vi "Splash screen.vi"(8 "error in (no error)":errorcluster) -> (0 "error out":errorcluster)   [LabVIEW 2016]
panel:
  out "String":string
  in  "Blank Button":bool
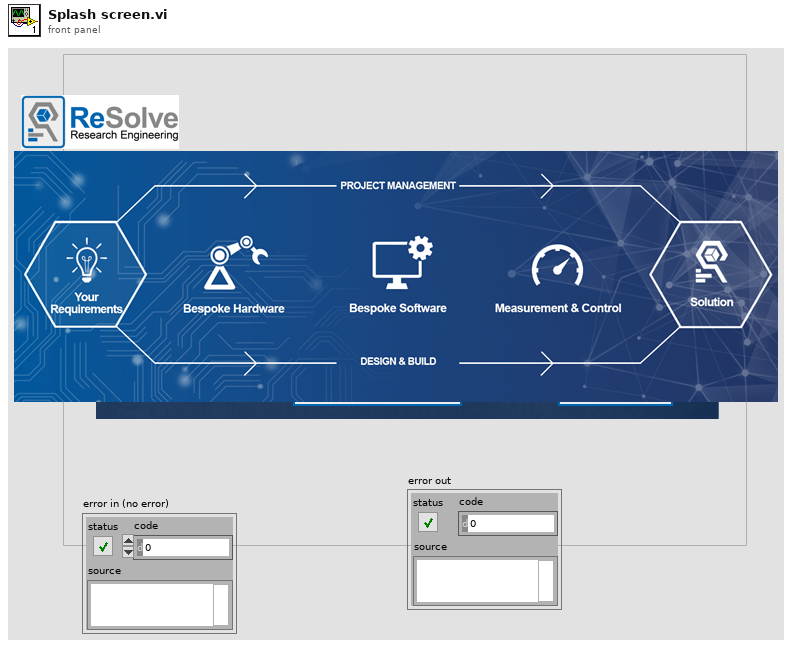
[diagram p1: front panel]
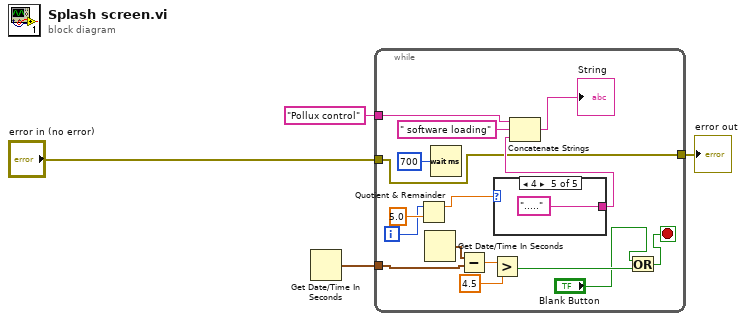
[diagram p0: block diagram]
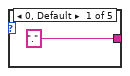
[diagram p2: hidden frame]
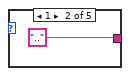
[diagram p3: hidden frame]
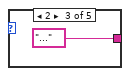
[diagram p4: hidden frame]
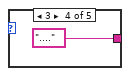
[diagram p5: hidden frame]
diagram:
  n1 = Get Date/Time In Seconds() -> (seconds since 1Jan1904=w4:timestamp)
  n2 = while {
    tunnel: "Pollux control" -> [w13]
    tunnel: w4 -> [w11]
    tunnel: "error in (no error)" -> [w6]
    tunnel: [w6] -> w3
    i -> [w16]
    stop <- w7 stop-if-true
    n3 = Quotient & Remainder(x=w16, y=5.0) -> (x-y*floor(x/y)=w15:dbl)  [unwired: 1 out]
    n4 = Get Date/Time In Seconds() -> (seconds since 1Jan1904=w12:timestamp)
    n5 = Wait (ms)(milliseconds to wait=u32 700) -> ()  [unwired: 1 out]
    n6 = Subtract(x=w12, y=w11) -> (x-y=w10:dbl)
    n7 = Greater?(x=w10, y=4.5) -> (0:w8:bool)
    n8 = case shown="4" w15 {
      tunnel: ["." ".." "..." "...." "....."] -> w14
      frame 0, Default {
      }
      frame 1 {
      }
      frame 2 {
      }
      frame 3 {
      }
      frame 4 {
      }
    }
    n9 = Concatenate Strings(w13, " software loading", w14) -> (→"String":string)
    n10 = Or(x="Blank Button", y=w8) -> (x .or. y?=w7:bool)
  }
  "error out" <- w3
